vi "attempt-circleFitOnFly.vi"() -> ()   [LabVIEW 2016]
uses:
  <vilib>/vision/Measure.llb/Edge Options.ctl
  <vilib>/vision/Measure.llb/Edge Polarity.ctl
  Motion/HomeMultiple.vi
panel:
  out "Error report":errorcluster
  in  "error in (no error)":errorcluster
  in  "Stop Stage":bool
  out "Moving":bool
  out "Homed":bool
  out "XYZ Stage Current Position":T1={"X [-750, 750 mm]"=-538.7066830444336, "Y [-150, 30 mm]"=-21.699673614501947, "Z [-50, 50 mm]"=3.7042}
  out "N moves":i32
  in  "Send stage to XYZ [mm]":T2
  in  "Axes Speeds [mm/s]":T3={"X Speed"=25.0, "Y Speed"=12.5, "Z Speed"=5.0}
  in  "Home stage":bool
  in  "Move stage":bool
  out "Fitted Circle (Find Circular Edge 1)":T4={"Center (Pixels)"={"X"=1382.2122, "Y"=1051.7542}, "Radius (Pixels)"=145.5667266845703, "Center (Real-World)"={"X"=4111.894, "Y"=-2284.6375}, "Radius (Real-World)"=484.9685191942223, "Roundness (Real-World)"=21.632436942481505, "Average Strength"=60.52941176470587, "Average SNR (dB)"=8.686059708305132} {"Average SNR (dB)" format="%.2f"; "Average Strength" format="%.2f"; "Roundness (Real-World)" format="%.2f"; "Radius (Real-World)" format="%.2f"; "Center (Real-World)"."Y" format="%.2f"; "Center (Real-World)"."X" format="%.2f"; "Radius (Pixels)" format="%.2f"; "Center (Pixels)"."Y" format="%.2f"; "Center (Pixels)"."X" format="%.2f"}
  out "ROI Pixel Statistics (Line Profile 1)":T5={"Min"=5.0, "Max"=255.0, "Mean"=78.77172, "Std Dev"=64.32993, "Count"=2567} {"Min" format="%.2f"; "Std Dev" format="%.2f"; "Mean" format="%.2f"; "Max" format="%.2f"}
  out "Line Profile":cluster{"x0":sgl, "dx":sgl, "Pixels Line":sgl[]}(graph)={"x0"=0.0, "dx"=1.0, "Pixels Line"=[40.0, 43.0, 37.0, 36.0, 39.0, 32.0, 31.0, 26.0, 24.0, 22.0, 19.0, 15.0, 14.0, 14.0, 15.0, 13.0, 11.0, 15.0, 9.0, 15.0, 15.0, 10.0, 9.0, 12.0, 9.0, 9.0, 11.0, 11.0, 10.0, 9.0, 8.0, 8.0, 6.0, 12.0, 9.0, 10.0, 10.0, 7.0, 9.0, 8.0, 12.0, 6.0, 12.0, 10.0, 7.0, 8.0, 7.0, 8.0, 9.0, 8.0, 7.0, 8.0, 10.0, 6.0, 8.0, 10.0, 5.0, 10.0, 8.0, 8.0, 6.0, 8.0, 8.0, 5.0, 7.0, 9.0, 7.0, 7.0, 10.0, 9.0, 8.0, 7.0, 8.0, 10.0, 6.0, 9.0, 9.0, 8.0, 11.0, 11.0, 10.0, 11.0, 12.0, 15.0, 15.0, 15.0, 18.0, 15.0, 19.0, 16.0, 21.0, 22.0, 19.0, 27.0, 23.0, 28.0, 28.0, 33.0, 34.0, 30.0, 42.0, 40.0, 43.0, 44.0, 45.0, 48.0, 48.0, 50.0, 45.0, 48.0, 52.0, 67.0, 57.0, 64.0, 63.0, 61.0, 62.0, 67.0, 65.0, 65.0, 65.0, 73.0, 64.0, 75.0, 74.0, 73.0, 79.0, 77.0, 84.0, 85.0, 87.0, 80.0, 88.0, 86.0, 85.0, 86.0, 91.0, 78.0, 85.0, 83.0, 99.0, 89.0, 95.0, 90.0, 94.0, 87.0, 98.0, 97.0, 99.0, 101.0, 100.0, 96.0, 94.0, 107.0, 106.0, 103.0, 116.0, 109.0, 112.0, 106.0, 105.0, 112.0, 107.0, 113.0, 120.0, 106.0, 114.0, 104.0, 116.0, 119.0, 117.0, 109.0, 117.0, 114.0, 114.0, 112.0, 119.0, 112.0, 117.0, 112.0, 116.0, 123.0, 111.0, 111.0, 115.0, 120.0, 97.0, 112.0, 110.0, 100.0, 113.0, 109.0, 110.0, 116.0, 116.0, 116.0, 112.0, 120.0, 125.0, 106.0, 126.0, 128.0, 113.0, 123.0, 100.0, 106.0, 119.0, 116.0, 123.0, 119.0, 113.0, 128.0, 125.0, 131.0, 133.0, 128.0, 134.0, 137.0, 128.0, 120.0, 122.0, 105.0, 118.0, 111.0, 110.0, 104.0, 105.0, 102.0, 112.0, 100.0, 107.0, 105.0, 114.0, 105.0, 116.0, 104.0, 104.0, 114.0, 106.0, 98.0, 96.0, 89.0, 94.0, 84.0, 88.0, 94.0, 99.0, 94.0, 100.0, 110.0, 112.0, 87.0, 100.0, 94.0, 102.0, 97.0, 107.0, 87.0, 90.0, 93.0, 101.0, 100.0, 104.0, 107.0, 110.0, 100.0, 111.0, 106.0, 104.0, 103.0, 108.0, 101.0, 98.0, 97.0, 98.0, 103.0, 95.0, 99.0, 100.0, 86.0, 97.0, 103.0, 102.0, 102.0, 105.0, 101.0, 102.0, 108.0, 104.0, 97.0, 99.0, 104.0, 103.0, 98.0, 97.0, 104.0, 109.0, 107.0, 109.0, 103.0, 114.0, 114.0, 112.0, 110.0, 102.0, 104.0, 100.0, 98.0, 104.0, 107.0, 107.0, 103.0, 107.0, 101.0, 107.0, 101.0, 105.0, 101.0, 107.0, 89.0, 86.0, 80.0, 79.0, 77.0, 80.0, 85.0, 84.0, 93.0, 88.0, 88.0, 86.0, 89.0, 98.0, 94.0, 93.0, 101.0, 94.0, 108.0, 106.0, 98.0, 106.0, 93.0, 101.0, 98.0, 88.0, 87.0, 85.0, 104.0, 92.0, 87.0, 84.0, 81.0, 89.0, 82.0, 86.0, 81.0, 80.0, 81.0, 84.0, 86.0, 89.0, 89.0, 86.0, 87.0, 86.0, 79.0, 79.0, 88.0, 83.0, 77.0, 84.0, 89.0, 84.0, 85.0, 80.0, 81.0, 80.0, 82.0, 89.0, 95.0, 88.0, 85.0, 90.0, 82.0, 92.0, 94.0, 100.0, 101.0, 89.0, 91.0, 105.0, 103.0, 99.0, 99.0, 100.0, 95.0, 94.0, 97.0, 110.0, 103.0, 103.0, 92.0, 91.0, 98.0, 98.0, 104.0, 95.0, 100.0, 107.0, 101.0, 110.0, 112.0, 104.0, 97.0, 108.0, 107.0, 109.0, 106.0, 116.0, 107.0, 99.0, 104.0, 114.0, 110.0, 109.0, 110.0, 110.0, 113.0, 101.0, 117.0, 108.0, 109.0, 120.0, 103.0, 105.0, 95.0, 91.0, 85.0, 89.0, 89.0, 81.0, 82.0, 79.0, 88.0, 89.0, 90.0, 97.0, 93.0, 104.0, 94.0, 99.0, 105.0, 110.0, 101.0, 97.0, 107.0, 110.0, 91.0, 107.0, 105.0, 119.0, 112.0, 112.0, 112.0, 121.0, 116.0, 131.0, 105.0, 116.0, 113.0, 126.0, 120.0, 115.0, 121.0, 114.0, 111.0, 119.0, 117.0, 121.0, 110.0, 101.0, 113.0, 109.0, 109.0, 111.0, 105.0, 107.0, 109.0, 109.0, 104.0, 107.0, 91.0, 102.0, 112.0, 105.0, 97.0, 103.0, 111.0, 98.0, 103.0, 106.0, 100.0, 111.0, 105.0, 111.0, 109.0, 111.0, 100.0, 104.0, 113.0, 107.0, 113.0, 110.0, 112.0, 95.0, 112.0, 99.0, 108.0, 106.0, 95.0, 98.0, 92.0, 93.0, 88.0, 93.0, 90.0, 88.0, 82.0, 81.0, 80.0, 83.0, 73.0, 78.0, 79.0, 91.0, 92.0, 91.0, 99.0, 105.0, 103.0, 106.0, 104.0, 114.0, 107.0, 101.0, 109.0, 106.0, 107.0, 101.0, 99.0, 98.0, 101.0, 112.0, 107.0, 97.0, 106.0, 108.0, 110.0, 112.0, 104.0, 104.0, 111.0, 103.0, 98.0, 109.0, 104.0, 103.0, 100.0, 104.0, 104.0, 104.0, 102.0, 104.0, 102.0, 104.0, 95.0, 93.0, 91.0, 87.0, 86.0, 88.0, 80.0, 77.0, 80.0, 76.0, 69.0, 69.0, 71.0, 79.0, 83.0, 89.0, 90.0, 86.0, 85.0, 85.0, 81.0, 77.0, 89.0, 85.0, 90.0, 98.0, 96.0, 97.0, 97.0, 105.0, 99.0, 97.0, 104.0, 105.0, 106.0, 101.0, 98.0, 104.0, 93.0, 104.0, 106.0, 101.0, 90.0, 94.0, 107.0, 99.0, 95.0, 92.0, 101.0, 101.0, 98.0, 100.0, 90.0, 92.0, 88.0, 97.0, 98.0, 100.0, 87.0, 101.0, 99.0, 86.0, 100.0, 88.0, 98.0, 97.0, 94.0, 97.0, 99.0, 100.0, 103.0, 98.0, 103.0, 114.0, 107.0, 102.0, 97.0, 99.0, 106.0, 109.0, 112.0, 103.0, 103.0, 103.0, 100.0, 95.0, 99.0, 100.0, 93.0, 94.0, 101.0, 93.0, 97.0, 98.0, 102.0, 95.0, 93.0, 93.0, 106.0, 100.0, 109.0, 98.0, 105.0, 96.0, 101.0, 102.0, 101.0, 92.0, 89.0, 92.0, 86.0, 99.0, 101.0, 94.0, 92.0, 95.0, 95.0, 93.0, 93.0, 92.0, 100.0, 94.0, 85.0, 85.0, 85.0, 85.0, 88.0, 81.0, 94.0, 88.0, 93.0, 100.0, 94.0, 92.0, 88.0, 92.0, 92.0, 95.0, 82.0, 85.0, 88.0, 84.0, 83.0, 94.0, 89.0, 93.0, 88.0, 87.0, 83.0, 91.0, 77.0, 81.0, 85.0, 77.0, 86.0, 89.0, 88.0, 84.0, 80.0, 79.0, 89.0, 89.0, 92.0, 84.0, 94.0, 82.0, 87.0, 90.0, 84.0, 84.0, 92.0, 80.0, 81.0, 71.0, 83.0, 85.0, 87.0, 90.0, 86.0, 93.0, 81.0, 88.0, 91.0, 89.0, 83.0, 95.0, 86.0, 95.0, 90.0, 86.0, 95.0, 84.0, 79.0, 82.0, 85.0, 84.0, 80.0, 82.0, 75.0, 80.0, 89.0, 90.0, 88.0, 85.0, 94.0, 91.0, 93.0, 94.0, 93.0, 88.0, 85.0, 91.0, 82.0, 92.0, 86.0, 84.0, 80.0, 81.0, 88.0, 85.0, 85.0, 93.0, 87.0, 97.0, 94.0, 97.0, 93.0, 97.0, 86.0, 106.0, 92.0, 94.0, 99.0, 101.0, 94.0, 96.0, 89.0, 92.0, 84.0, 89.0, 91.0, 95.0, 103.0, 92.0, 106.0, 104.0, 107.0, 112.0, 97.0, 104.0, 101.0, 104.0, 107.0, 88.0, 91.0, 100.0, 101.0, 102.0, 98.0, 104.0, 104.0, 101.0, 97.0, 98.0, 85.0, 89.0, 98.0, 100.0, 94.0, 95.0, 97.0, 86.0, 95.0, 92.0, 91.0, 98.0, 98.0, 105.0, 94.0, 101.0, 97.0, 88.0, 96.0, 103.0, 109.0, 104.0, 94.0, 88.0, 101.0, 106.0, 93.0, 102.0, 97.0, 95.0, 91.0, 95.0, 87.0, 94.0, 92.0, 101.0, 96.0, 92.0, 93.0, 91.0, 90.0, 92.0, 90.0, 97.0, 95.0, 100.0, 94.0, 106.0, 97.0, 103.0, 94.0, 94.0, 92.0, 101.0, 91.0, 97.0, 85.0, 90.0, 83.0, 83.0, 82.0, 78.0, 73.0, 75.0, 79.0, 74.0, 77.0, 79.0, 78.0, 75.0, 73.0, 77.0, 80.0, 76.0, 69.0, 73.0, 68.0, 70.0, 60.0, 64.0, 55.0, 59.0, 56.0, 53.0, 49.0, 40.0, 39.0, 39.0, 35.0, 28.0, 28.0, 27.0, 23.0, 22.0, 22.0, 25.0, 21.0, 26.0, 19.0, 23.0, 21.0, 21.0, 24.0, 25.0, 22.0, 28.0, 20.0, 18.0, 24.0, 18.0, 18.0, 20.0, 15.0, 16.0, 15.0, 14.0, 13.0, 13.0, 11.0, 13.0, 15.0, 14.0, 18.0, 16.0, 19.0, 15.0, 19.0, 19.0, 18.0, 15.0, 22.0, 15.0, 16.0, 15.0, 16.0, 15.0, 19.0, 16.0, 14.0, 18.0, 16.0, 15.0, 15.0, 15.0, 17.0, 12.0, 18.0, 13.0, 16.0, 12.0, 14.0, 15.0, 10.0, 13.0, 20.0, 15.0, 12.0, 16.0, 18.0, 16.0, 16.0, 17.0, 12.0, 19.0, 15.0, 15.0, 15.0, 13.0, 13.0, 12.0, 15.0, 15.0, 15.0, 17.0, 14.0, 12.0, 15.0, 16.0, 21.0, 11.0, 12.0, 14.0, 17.0, 13.0, 11.0, 17.0, 15.0, 17.0, 17.0, 12.0, 15.0, 18.0, 13.0, 15.0, 17.0, 16.0, 18.0, 17.0, 10.0, 16.0, 16.0, 16.0, 19.0, 14.0, 16.0, 20.0, 14.0, 16.0, 17.0, 15.0, 15.0, 18.0, 16.0, 13.0, 17.0, 13.0, 15.0, 13.0, 21.0, 12.0, 15.0, 14.0, 15.0, 15.0, 15.0, 18.0, 14.0, 14.0, 13.0, 16.0, 16.0, 17.0, 17.0, 15.0, 16.0, 15.0, 15.0, 18.0, 16.0, 15.0, 14.0, 19.0, 16.0, 10.0, 18.0, 13.0, 14.0, 15.0, 15.0, 16.0, 13.0, 15.0, 16.0, 15.0, 13.0, 13.0, 15.0, 14.0, 19.0, 16.0, 17.0, 11.0, 13.0, 12.0, 15.0, 17.0, 20.0, 19.0, 15.0, 22.0, 16.0, 16.0, 15.0, 16.0, 19.0, 15.0, 17.0, 17.0, 15.0, 15.0, 14.0, 16.0, 15.0, 11.0, 17.0, 19.0, 17.0, 14.0, 15.0, 18.0, 18.0, 14.0, 17.0, 18.0, 17.0, 16.0, 18.0, 13.0, 17.0, 18.0, 15.0, 12.0, 20.0, 17.0, 15.0, 16.0, 19.0, 17.0, 21.0, 13.0, 15.0, 20.0, 16.0, 16.0, 17.0, 18.0, 16.0, 21.0, 16.0, 16.0, 19.0, 19.0, 20.0, 16.0, 22.0, 19.0, 20.0, 16.0, 18.0, 16.0, 19.0, 17.0, 22.0, 18.0, 15.0, 18.0, 19.0, 15.0, 21.0, 17.0, 17.0, 19.0, 19.0, 21.0, 15.0, 21.0, 17.0, 24.0, 18.0, 20.0, 17.0, 17.0, 21.0, 19.0, 17.0, 19.0, 21.0, 18.0, 21.0, 17.0, 18.0, 28.0, 24.0, 24.0, 22.0, 29.0, 36.0, 39.0, 49.0, 52.0, 66.0, 99.0, 142.0, 181.0, 219.0, 214.0, 193.0, 195.0, 163.0, 173.0, 193.0, 230.0, 246.0, 255.0, 255.0, 255.0, 255.0, 255.0, 255.0, 255.0, 255.0, 255.0, 255.0, 255.0, 255.0, 255.0, 255.0, 255.0, 255.0, 255.0, 248.0, 240.0, 222.0, 220.0, 211.0, 219.0, 212.0, 219.0, 219.0, 216.0, 217.0, 207.0, 216.0, 228.0, 215.0, 227.0, 211.0, 226.0, 221.0, 207.0, 222.0, 245.0, 239.0, 253.0, 255.0, 255.0, 255.0, 255.0, 255.0, 255.0, 255.0, 255.0, 255.0, 255.0, 255.0, 255.0, 255.0, 255.0, 255.0, 255.0, 255.0, 255.0, 255.0, 255.0, 255.0, 255.0, 255.0, 255.0, 255.0, 255.0, 255.0, 255.0, 255.0, 255.0, 255.0, 255.0, 255.0, 255.0, 255.0, 255.0, 255.0, 255.0, 255.0, 255.0, 255.0, 255.0, 240.0, 198.0, 182.0, 179.0, 193.0, 200.0, 216.0, 202.0, 196.0, 199.0, 195.0, 210.0, 214.0, 253.0, 255.0, 255.0, 255.0, 255.0, 255.0, 255.0, 248.0, 234.0, 251.0, 255.0, 255.0, 255.0, 255.0, 255.0, 255.0, 255.0, 255.0, 255.0, 255.0, 255.0, 255.0, 255.0, 255.0, 252.0, 217.0, 205.0, 207.0, 233.0, 217.0, 230.0, 239.0, 228.0, 211.0, 199.0, 207.0, 205.0, 213.0, 215.0, 217.0, 217.0, 204.0, 229.0, 232.0, 230.0, 222.0, 233.0, 254.0, 255.0, 255.0, 255.0, 244.0, 233.0, 206.0, 229.0, 194.0, 205.0, 197.0, 179.0, 187.0, 185.0, 205.0, 223.0, 239.0, 246.0, 255.0, 255.0, 255.0, 255.0, 254.0, 230.0, 216.0, 197.0, 192.0, 210.0, 181.0, 198.0, 192.0, 202.0, 212.0, 226.0, 247.0, 240.0, 229.0, 223.0, 233.0, 255.0, 255.0, 255.0, 247.0, 230.0, 216.0, 218.0, 226.0, 255.0, 255.0, 253.0, 255.0, 255.0, 237.0, 247.0, 244.0, 248.0, 255.0, 255.0, 255.0, 255.0, 250.0, 243.0, 220.0, 215.0, 218.0, 226.0, 242.0, 255.0, 255.0, 255.0, 255.0, 255.0, 255.0, 255.0, 255.0, 255.0, 255.0, 255.0, 255.0, 248.0, 255.0, 255.0, 255.0, 210.0, 190.0, 166.0, 158.0, 163.0, 189.0, 200.0, 214.0, 207.0, 192.0, 201.0, 199.0, 190.0, 172.0, 165.0, 166.0, 176.0, 171.0, 192.0, 189.0, 178.0, 162.0, 168.0, 166.0, 178.0, 181.0, 191.0, 190.0, 178.0, 162.0, 167.0, 163.0, 173.0, 162.0, 163.0, 157.0, 159.0, 158.0, 158.0, 159.0, 174.0, 190.0, 190.0, 209.0, 217.0, 230.0, 252.0, 244.0, 247.0, 232.0, 223.0, 210.0, 179.0, 175.0, 128.0, 99.0, 58.0, 49.0, 38.0, 33.0, 28.0, 23.0, 23.0, 31.0, 19.0, 27.0, 18.0, 17.0, 18.0, 15.0, 21.0, 18.0, 15.0, 18.0, 16.0, 15.0, 17.0, 14.0, 18.0, 22.0, 14.0, 16.0, 19.0, 13.0, 18.0, 18.0, 14.0, 14.0, 14.0, 16.0, 16.0, 16.0, 16.0, 15.0, 17.0, 14.0, 19.0, 15.0, 17.0, 17.0, 16.0, 15.0, 12.0, 19.0, 19.0, 19.0, 18.0, 12.0, 20.0, 17.0, 16.0, 13.0, 15.0, 17.0, 16.0, 19.0, 17.0, 15.0, 15.0, 14.0, 19.0, 13.0, 20.0, 19.0, 18.0, 23.0, 15.0, 12.0, 17.0, 20.0, 13.0, 14.0, 13.0, 12.0, 16.0, 18.0, 17.0, 19.0, 19.0, 17.0, 13.0, 18.0, 18.0, 16.0, 16.0, 19.0, 17.0, 18.0, 18.0, 18.0, 13.0, 17.0, 14.0, 16.0, 14.0, 15.0, 11.0, 12.0, 16.0, 15.0, 11.0, 16.0, 16.0, 17.0, 16.0, 12.0, 20.0, 16.0, 16.0, 16.0, 15.0, 15.0, 13.0, 19.0, 16.0, 15.0, 11.0, 17.0, 15.0, 20.0, 8.0, 15.0, 16.0, 19.0, 16.0, 16.0, 14.0, 17.0, 16.0, 20.0, 15.0, 20.0, 18.0, 15.0, 17.0, 21.0, 20.0, 16.0, 21.0, 20.0, 21.0, 17.0, 23.0, 18.0, 15.0, 13.0, 15.0, 12.0, 9.0, 14.0, 14.0, 15.0, 11.0, 13.0, 12.0, 14.0, 13.0, 17.0, 15.0, 13.0, 12.0, 12.0, 18.0, 16.0, 13.0, 11.0, 16.0, 18.0, 14.0, 16.0, 17.0, 15.0, 12.0, 16.0, 18.0, 16.0, 14.0, 18.0, 15.0, 19.0, 13.0, 13.0, 18.0, 13.0, 13.0, 14.0, 12.0, 12.0, 14.0, 16.0, 15.0, 13.0, 14.0, 13.0, 11.0, 15.0, 15.0, 19.0, 18.0, 18.0, 15.0, 16.0, 17.0, 15.0, 15.0, 18.0, 13.0, 16.0, 18.0, 18.0, 17.0, 16.0, 19.0, 29.0, 29.0, 41.0, 52.0, 61.0, 65.0, 84.0, 92.0, 89.0, 101.0, 101.0, 99.0, 112.0, 113.0, 104.0, 107.0, 113.0, 116.0, 114.0, 114.0, 113.0, 120.0, 130.0, 136.0, 153.0, 162.0, 164.0, 174.0, 183.0, 181.0, 171.0, 168.0, 168.0, 163.0, 148.0, 149.0, 138.0, 132.0, 126.0, 127.0, 107.0, 117.0, 113.0, 120.0, 119.0, 114.0, 100.0, 110.0, 100.0, 107.0, 111.0, 98.0, 97.0, 97.0, 88.0, 87.0, 91.0, 95.0, 85.0, 88.0, 90.0, 86.0, 83.0, 84.0, 81.0, 82.0, 82.0, 85.0, 88.0, 87.0, 79.0, 68.0, 67.0, 64.0, 72.0, 68.0, 68.0, 75.0, 70.0, 88.0, 76.0, 87.0, 75.0, 81.0, 77.0, 90.0, 85.0, 89.0, 99.0, 92.0, 96.0, 95.0, 109.0, 94.0, 86.0, 93.0, 86.0, 80.0, 83.0, 86.0, 90.0, 94.0, 89.0, 97.0, 95.0, 104.0, 97.0, 107.0, 101.0, 101.0, 94.0, 92.0, 100.0, 95.0, 94.0, 89.0, 95.0, 83.0, 87.0, 88.0, 76.0, 83.0, 92.0, 93.0, 93.0, 95.0, 98.0, 97.0, 99.0, 89.0, 96.0, 97.0, 93.0, 94.0, 96.0, 85.0, 92.0, 92.0, 87.0, 99.0, 93.0, 90.0, 96.0, 98.0, 88.0, 92.0, 97.0, 99.0, 98.0, 92.0, 91.0, 86.0, 87.0, 100.0, 93.0, 86.0, 87.0, 83.0, 75.0, 80.0, 73.0, 62.0, 73.0, 65.0, 67.0, 68.0, 79.0, 74.0, 70.0, 75.0, 70.0, 72.0, 65.0, 65.0, 66.0, 67.0, 69.0, 73.0, 74.0, 69.0, 76.0, 79.0, 71.0, 74.0, 72.0, 79.0, 76.0, 74.0, 72.0, 74.0, 71.0, 68.0, 71.0, 71.0, 85.0, 85.0, 81.0, 88.0, 79.0, 84.0, 84.0, 80.0, 80.0, 83.0, 85.0, 80.0, 89.0, 97.0, 92.0, 83.0, 84.0, 92.0, 82.0, 81.0, 91.0, 85.0, 83.0, 89.0, 82.0, 93.0, 85.0, 86.0, 89.0, 86.0, 87.0, 76.0, 79.0, 80.0, 72.0, 77.0, 70.0, 76.0, 85.0, 80.0, 74.0, 73.0, 80.0, 73.0, 82.0, 64.0, 71.0, 64.0, 64.0, 68.0, 67.0, 71.0, 63.0, 75.0, 67.0, 71.0, 67.0, 62.0, 66.0, 60.0, 67.0, 68.0, 63.0, 69.0, 68.0, 67.0, 68.0, 58.0, 67.0, 64.0, 58.0, 61.0, 58.0, 54.0, 60.0, 62.0, 68.0, 58.0, 62.0, 57.0, 64.0, 71.0, 70.0, 68.0, 68.0, 63.0, 73.0, 73.0, 65.0, 55.0, 52.0, 45.0, 40.0, 42.0, 48.0, 52.0, 53.0, 51.0, 56.0, 56.0, 56.0, 51.0, 53.0, 61.0, 59.0, 54.0, 51.0, 46.0, 44.0, 45.0, 50.0, 47.0, 50.0, 44.0, 47.0, 57.0, 54.0, 58.0, 55.0, 68.0, 57.0, 72.0, 62.0, 61.0, 65.0, 73.0, 65.0, 67.0, 69.0, 71.0, 71.0, 73.0, 62.0, 69.0, 67.0, 66.0, 69.0, 64.0, 70.0, 69.0, 73.0, 81.0, 71.0, 77.0, 77.0, 67.0, 72.0, 75.0, 72.0, 72.0, 74.0, 76.0, 72.0, 81.0, 74.0, 74.0, 87.0, 79.0, 65.0, 83.0, 70.0, 77.0, 70.0, 74.0, 74.0, 86.0, 79.0, 73.0, 70.0, 64.0, 69.0, 70.0, 79.0, 75.0, 77.0, 68.0, 71.0, 64.0, 64.0, 77.0, 74.0, 69.0, 72.0, 73.0, 64.0, 64.0, 66.0, 60.0, 66.0, 66.0, 62.0, 64.0, 64.0, 68.0, 64.0, 62.0, 64.0, 64.0, 67.0, 70.0, 63.0, 60.0, 67.0, 63.0, 65.0, 67.0, 72.0, 64.0, 67.0, 67.0, 64.0, 54.0, 57.0, 53.0, 62.0, 62.0, 64.0, 68.0, 64.0, 70.0, 65.0, 79.0, 76.0, 71.0, 68.0, 66.0, 50.0, 46.0, 45.0, 39.0, 46.0, 40.0, 44.0, 46.0, 48.0, 59.0, 55.0, 58.0, 56.0, 58.0, 60.0, 55.0, 52.0, 56.0, 54.0, 55.0, 54.0, 59.0, 57.0, 70.0, 71.0, 79.0, 69.0, 60.0, 56.0, 56.0, 49.0, 40.0, 36.0, 44.0, 41.0, 37.0, 33.0, 43.0, 41.0, 56.0, 57.0, 52.0, 50.0, 47.0, 45.0, 43.0, 51.0, 50.0, 47.0, 56.0, 55.0, 53.0, 55.0, 49.0, 52.0, 53.0, 55.0, 48.0, 55.0, 48.0, 46.0, 51.0, 55.0, 56.0, 60.0, 53.0, 39.0, 36.0, 39.0, 36.0, 37.0, 34.0, 32.0, 35.0, 33.0, 32.0, 37.0, 43.0, 39.0, 44.0, 44.0, 43.0, 42.0, 44.0, 46.0, 42.0, 37.0, 39.0, 36.0, 38.0, 31.0, 34.0, 30.0, 34.0, 31.0, 35.0, 40.0, 34.0, 31.0, 32.0, 31.0, 34.0, 30.0, 38.0, 34.0, 32.0, 33.0, 34.0, 33.0, 39.0, 33.0, 39.0, 36.0, 33.0, 27.0, 25.0, 25.0, 22.0, 20.0, 28.0, 26.0, 31.0, 29.0, 32.0, 37.0, 36.0, 30.0, 24.0, 25.0, 30.0, 21.0, 23.0, 27.0, 22.0, 25.0, 27.0, 27.0, 29.0, 26.0, 22.0, 29.0, 28.0, 23.0, 26.0, 27.0, 28.0, 27.0, 31.0, 24.0, 25.0, 30.0, 34.0, 29.0, 28.0, 31.0, 31.0, 31.0, 32.0, 39.0, 34.0, 33.0, 27.0, 24.0, 22.0, 22.0, 23.0, 21.0, 29.0, 27.0, 30.0, 24.0, 23.0, 28.0, 23.0, 31.0, 29.0, 28.0, 27.0, 27.0, 25.0, 27.0, 33.0, 40.0, 32.0, 36.0, 35.0, 35.0, 31.0, 24.0, 31.0, 21.0, 25.0, 23.0, 24.0, 28.0, 24.0, 21.0, 25.0, 26.0, 25.0, 32.0, 30.0, 37.0, 39.0, 40.0, 39.0, 36.0, 28.0, 25.0, 22.0, 22.0, 26.0, 26.0, 25.0, 25.0, 27.0, 28.0, 32.0, 30.0, 31.0, 28.0, 36.0, 37.0, 34.0, 36.0, 34.0, 36.0, 32.0, 30.0, 31.0, 27.0, 27.0, 24.0, 27.0, 22.0, 24.0, 27.0, 24.0, 30.0, 33.0, 29.0, 26.0, 30.0, 31.0, 26.0, 31.0, 28.0, 32.0, 24.0, 27.0, 33.0, 25.0, 28.0, 33.0, 35.0, 36.0, 34.0, 25.0, 24.0, 24.0, 25.0, 24.0, 28.0, 24.0, 33.0, 27.0, 29.0, 30.0, 26.0, 29.0, 29.0, 30.0, 28.0, 26.0, 22.0, 19.0, 30.0, 29.0, 24.0, 21.0, 25.0, 25.0, 30.0, 24.0, 21.0, 19.0, 25.0, 22.0, 18.0, 24.0, 19.0, 23.0, 19.0, 20.0, 19.0, 18.0, 22.0, 21.0, 17.0, 19.0, 20.0, 18.0, 18.0, 18.0, 19.0, 17.0, 19.0, 13.0, 19.0, 13.0, 22.0, 19.0, 19.0, 18.0, 16.0, 19.0, 18.0, 21.0, 17.0, 19.0, 21.0, 16.0, 19.0, 16.0, 19.0, 20.0, 18.0, 16.0, 14.0, 15.0, 20.0, 19.0, 16.0, 19.0, 19.0, 15.0, 22.0, 20.0, 18.0, 20.0, 23.0, 18.0, 22.0, 21.0, 18.0, 22.0, 23.0, 19.0, 24.0, 22.0, 22.0, 25.0, 23.0, 23.0, 19.0, 21.0, 21.0, 27.0, 28.0, 30.0, 27.0, 31.0, 28.0, 24.0, 25.0, 28.0, 30.0, 36.0, 36.0, 32.0, 31.0, 28.0, 34.0, 31.0, 35.0, 36.0, 37.0, 35.0, 39.0, 30.0, 30.0, 33.0, 29.0, 31.0, 34.0, 37.0, 38.0, 44.0, 35.0, 39.0, 34.0, 34.0, 37.0, 30.0, 39.0, 30.0, 35.0, 30.0, 32.0, 34.0, 33.0, 35.0, 35.0, 34.0, 30.0, 36.0, 30.0, 30.0, 25.0, 23.0, 24.0, 22.0, 18.0, 20.0, 15.0, 15.0, 13.0, 10.0, 11.0, 10.0, 8.0, 8.0, 5.0, 8.0, 6.0, 5.0]}
  in  "Circle Fit Options":T6={"Process"=enum."Get First Edge", "Step Size"=10, "Max Pixel Radius"=3}
  in  "Options (Find Circular Edge 1)":T9={"Search  Direction"=0, "Edge Options"={"Edge Polarity"=0, "Kernel Size"=3, "Width"=3, "Minimum Edge Strength"=50.0, "Interpolation Type"=enum."Bilinear Fixed", "Data Processing Method"=enum."Average"}, "Show Search Area"=TRUE, "Show Search Lines"=TRUE, "Show Edges Found"=TRUE, "Show Result"=TRUE, "Search Area Color"=65280, "Search Lines Color"=255, "Edge Locations Color"=16776960, "Result Color"=16711680, "Overlay Group Name"=""} {"Search  Direction" items=["Outside to Inside", "Inside to Outside"]; "Edge Options"."Edge Polarity" items=["All Edges", "Rising Edges", "Falling Edges"]; "Edge Options"."Minimum Edge Strength" format="%.2f"; "Edge Options"."Width" step=2; "Edge Options"."Kernel Size" step=2}
  out "Image Number":u32=372
  in  "Stop Camera":bool
  out "Image Out":T10(plugin-control)
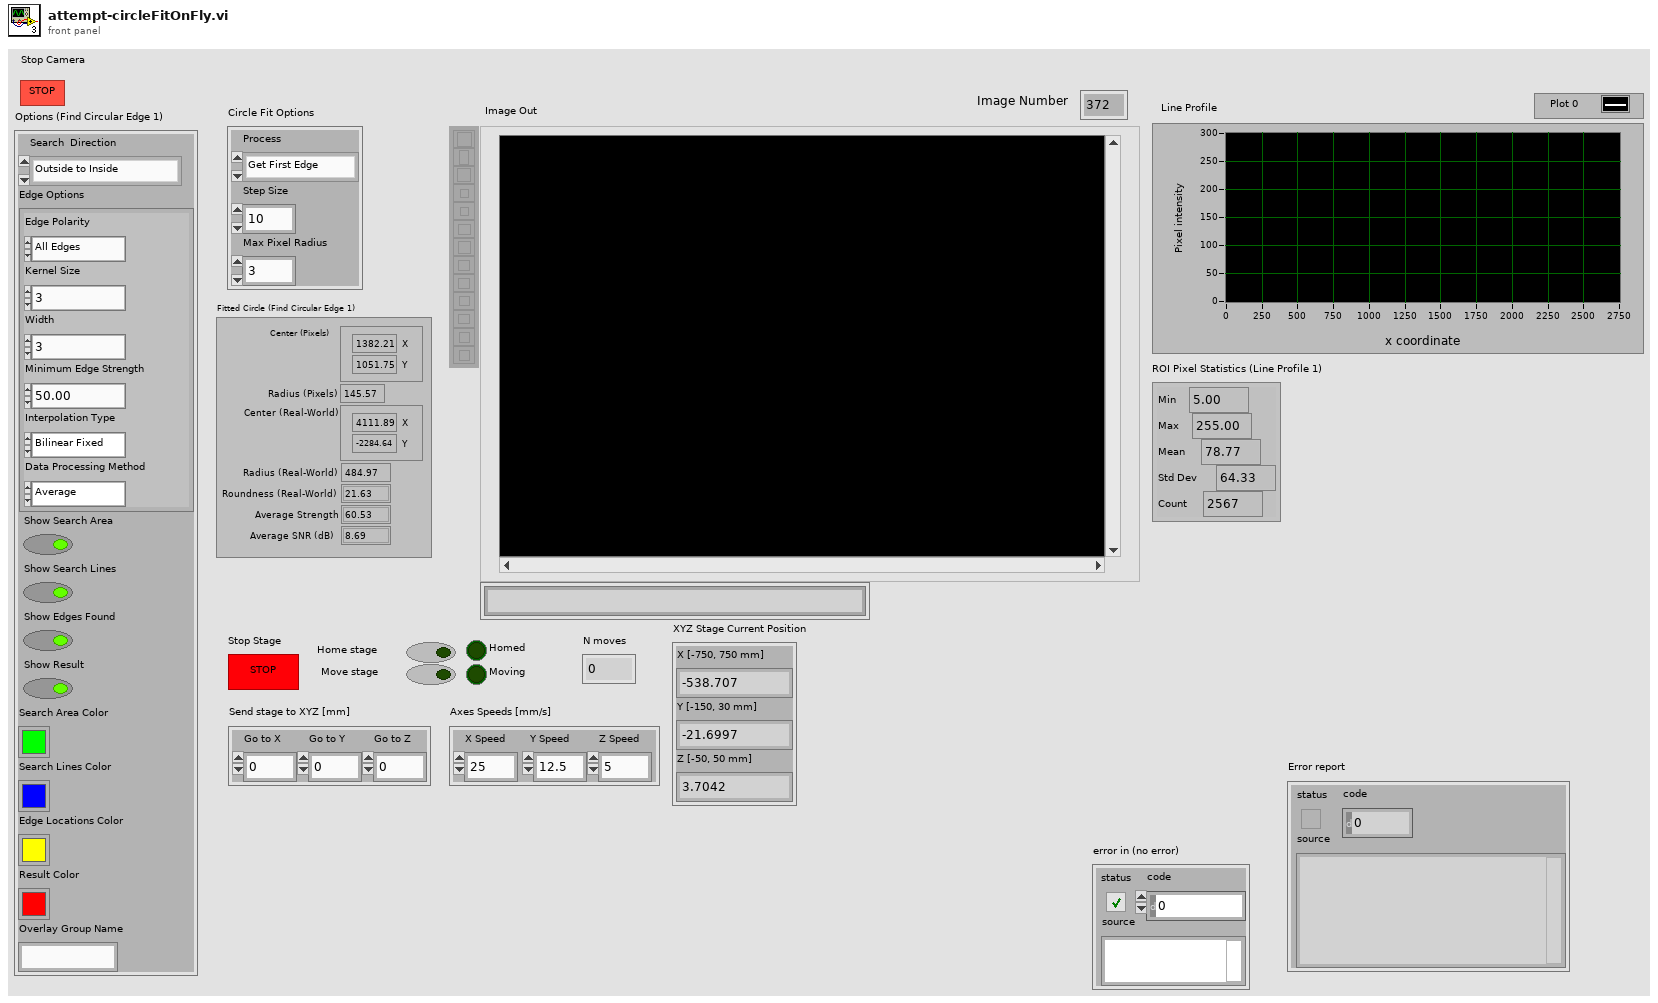
[diagram p1: front panel]
types:
  T1 = cluster{"X [-750, 750 mm]":dbl, "Y [-150, 30 mm]":dbl, "Z [-50, 50 mm]":dbl}
  T2 = cluster{"Go to X":dbl, "Go to Y":dbl, "Go to Z":dbl}
  T3 = cluster{"X Speed":dbl, "Y Speed":dbl, "Z Speed":dbl}
  T4 = cluster{"Center (Pixels)":cluster{"X":sgl, "Y":sgl}, "Radius (Pixels)":dbl, "Center (Real-World)":cluster{"X":sgl, "Y":sgl}, "Radius (Real-World)":dbl, "Roundness (Real-World)":dbl, "Average Strength":dbl, "Average SNR (dB)":dbl}
  T5 = cluster{"Min":sgl, "Max":sgl, "Mean":sgl, "Std Dev":sgl, "Count":i32}
  T6 = cluster{"Process":enum16{"Get First Edge", "Get First + Last Edge", "Get All Edges", "Get Best Edge"}, "Step Size":i32, "Max Pixel Radius":i32}
  T7 = typedef "Edge Options.ctl" = cluster{"Edge Polarity":T8, "Kernel Size":u32, "Width":u32, "Minimum Edge Strength":sgl, "Interpolation Type":enum32{"Zero Order", "Bilinear", "Quadratic", "Cubic", "Bilinear Fixed"}, "Data Processing Method":enum32{"Average", "Median"}}
  T8 = typedef "Edge Polarity.ctl" = u32
  T9 = cluster{"Search  Direction":u32, "Edge Options":T7, "Show Search Area":bool, "Show Search Lines":bool, "Show Edges Found":bool, "Show Result":bool, "Search Area Color":u32, "Search Lines Color":u32, "Edge Locations Color":u32, "Result Color":u32, "Overlay Group Name":string}
  T10 = typedef "IMAQ Image.ctl" = refnum<image>
  T11 = cluster{"Program Position Feedback":dbl, "Program Position Feedback 2":dbl, "Program Position Feedback 3":dbl}
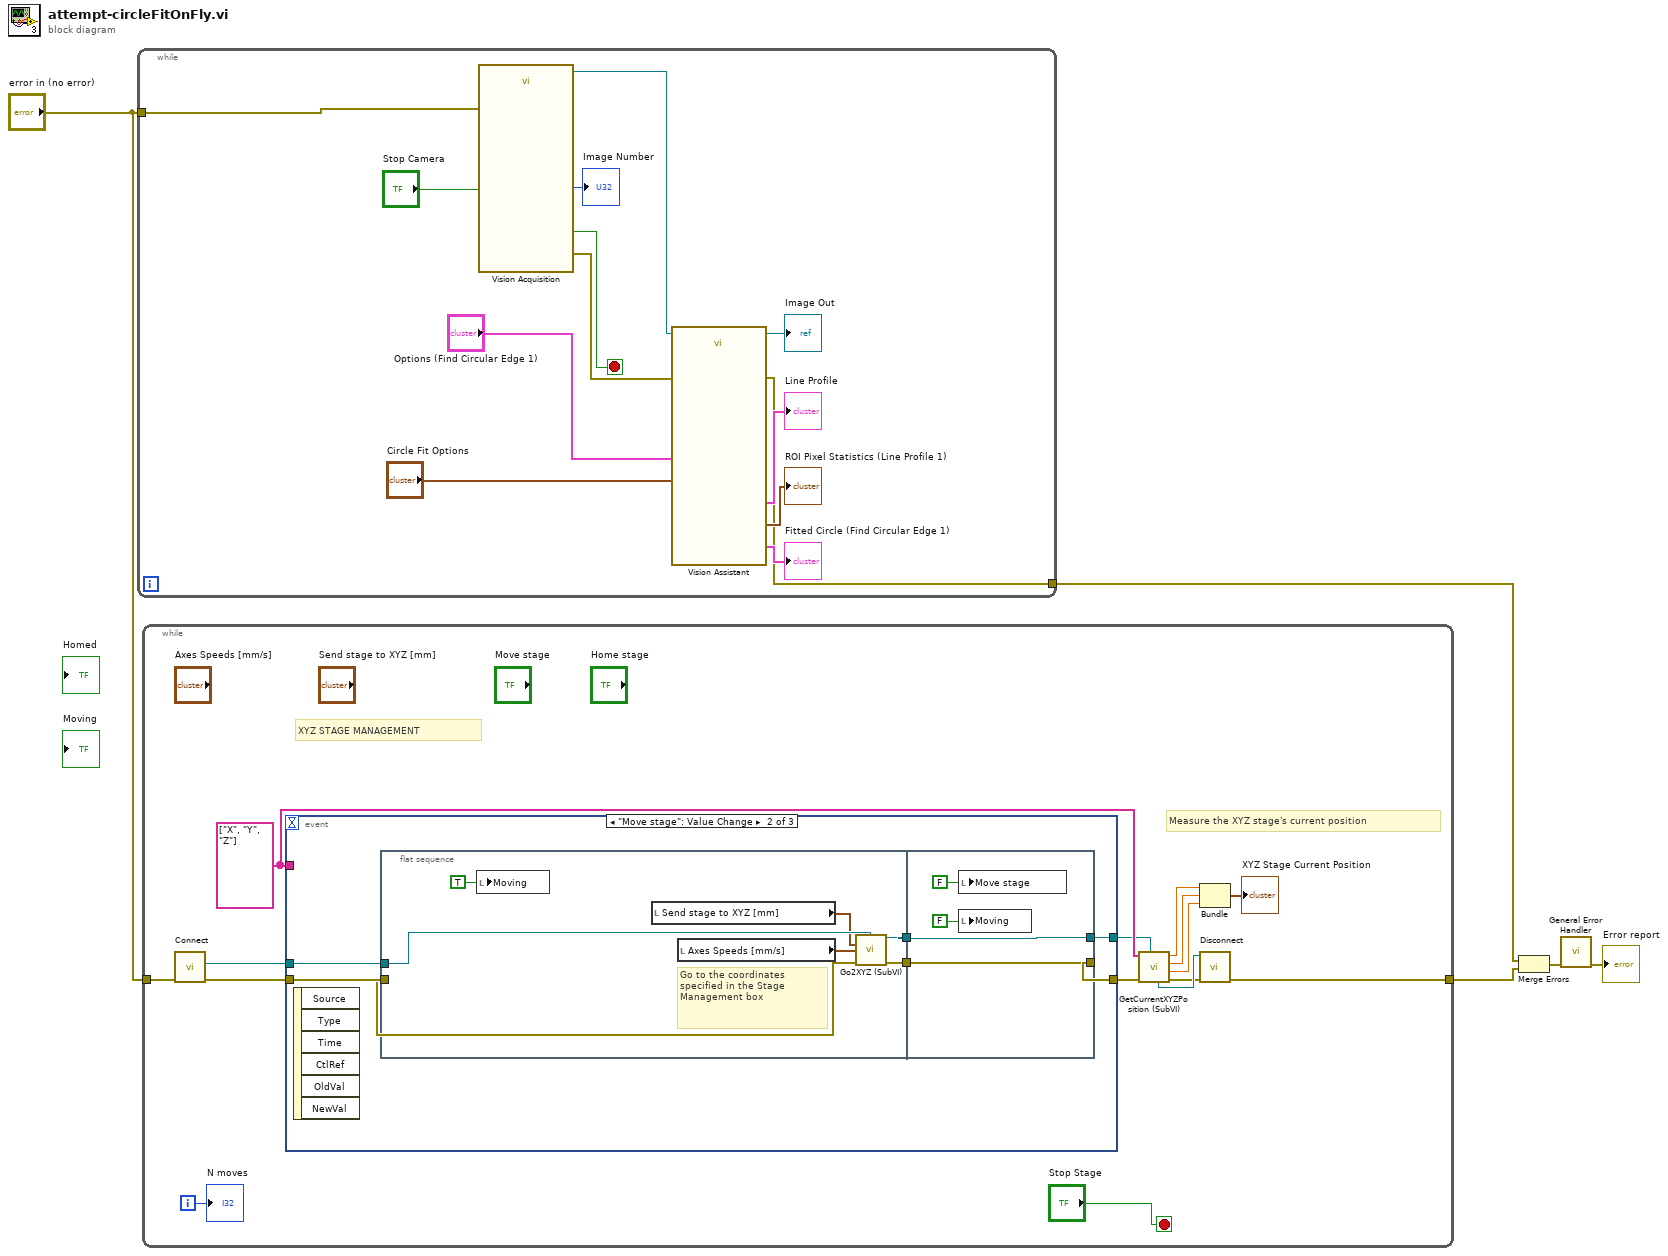
[diagram p0: block diagram]
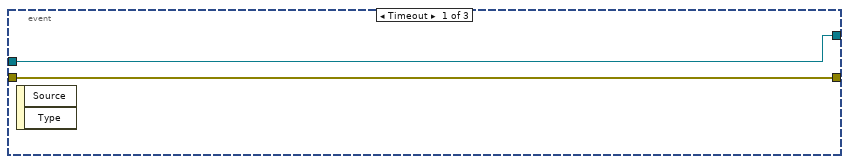
[diagram p2: hidden frame]
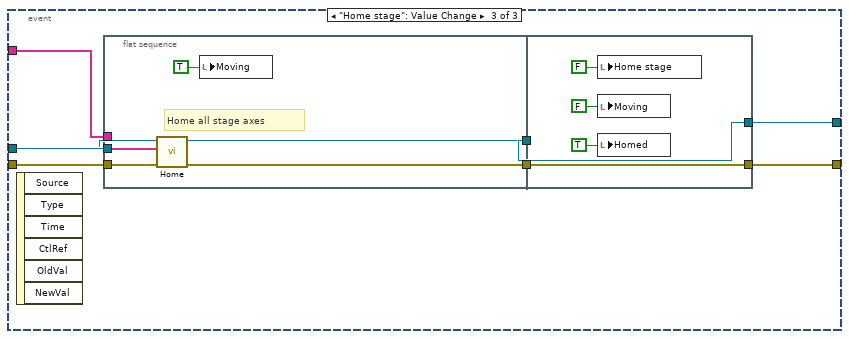
[diagram p3: hidden frame]
diagram:
  n1 = while {
    tunnel: "error in (no error)" -> [w8]
    tunnel: [w6] -> w3
    stop <- w17 stop-if-true
    n2 = call "Vision Acquisition"("Stop (F)"="Stop Camera", "error in"=w8) -> ("Image Out"=w15:T10, "Image Number"=→"Image Number":u32, "Stopped"=w17:bool, "error out"=w7:errorcluster)  [unwired: 21 in, 1 out]
    n3 = call "Vision Assistant"("Image In"=w15, "Options (Find Circular Edge 1)"="Options (Find Circular Edge 1)", "Circle Fit Options (Find Circular Edge 1)"="Circle Fit Options", "error in"=w7) -> ("Image Out"=→"Image Out":T10, "Line Profile (Line Profile 1)"=→"Line Profile":cluster{"x0":sgl, "dx":sgl, "Pixels Line":sgl[]}, "ROI Pixel Statistics (Line Profile 1)"=→"ROI Pixel Statistics (Line Profile 1)":T5, "Fitted Circle (Find Circular Edge 1)"=→"Fitted Circle (Find Circular Edge 1)":T4, "error out"=w6:errorcluster)  [unwired: 19 in]
  }
  n4 = while {
    tunnel: "error in (no error)" -> [w33]
    tunnel: [w20] -> w1
    i -> [w23]
    stop <- "Stop Stage" stop-if-true
    w24 = string[] ["X", "Y", "Z"] ("Axes Names")
    # "XYZ STAGE MANAGEMENT"
    # "Measure the XYZ stage's current position"
    n5 = call "Connect.vi"("error in (no error)"=w33) -> ("error out"=w31:errorcluster, "controller"=w32:refnum<k24>)  [unwired: 9 in]
    n6 = event shown="[1] \"Move stage\": Value Change" {
      selector: _ -> [_ _ _]
      dyn-events: _ -> [_ _ _]
      timeout: _ -> [_ _ _]
      tunnel: w32 -> [w35 w41 w59]
      tunnel: w31 -> [w34 w38 w58]
      tunnel: [w35 w40 w56] -> w22
      tunnel: [w34 w39 w57] -> w25
      tunnel: w24 -> [_ _ w55]
      event Timeout {
        n7 = event-data() -> ()  [unwired: 1 in, 2 out]
      }
      event "Move stage": Value Change {
        n8 = event-data() -> ()  [unwired: 1 in, 6 out]
        n9 = flat-sequence {
          tunnel: w41 -> [w48]
          tunnel: w38 -> [w45]
          tunnel: [w47] -> w37
          tunnel: [w46] -> w36
          tunnel: [w51] -> w39
          tunnel: [w52] -> w40
          tunnel: w37 -> [w52]
          tunnel: w36 -> [w51]
          frame #0 {
            # "Go to the coordinates\nspecified in the Stage\nManagement box"
            n10 = local write "Moving"(TRUE ("Moving")) -> ()
            n11 = local read "Send stage to XYZ [mm]"() -> (w43:T2)
            n12 = local read "Axes Speeds [mm/s]"() -> (w42:T3)
            n13 = call "Go2XYZ (SubVI).vi"(".NET Refnum in"=w48, "Go to Coordinates"=w43, "Axis Speeds"=w42, "error in (no error)"=w45) -> (".NET Refnum out"=w47:refnum<k24>, "error out"=w46:errorcluster)  [unwired: 8 in, 2 out]
          }
          frame #1 {
            n14 = local write "Move stage"(FALSE ("Move stage")) -> ()
            n15 = local write "Moving"(FALSE ("Moving")) -> ()
          }
        }
      }
      event "Home stage": Value Change {
        n16 = event-data() -> ()  [unwired: 1 in, 6 out]
        n17 = flat-sequence {
          tunnel: w59 -> [w65]
          tunnel: w58 -> [w64]
          tunnel: w55 -> [w61]
          tunnel: [w63] -> w54
          tunnel: [w62] -> w53
          tunnel: [w69] -> w56
          tunnel: [w70] -> w57
          tunnel: w54 -> [w70]
          tunnel: w53 -> [w69]
          frame #0 {
            # "Home all stage axes"
            n18 = call-poly "Home.vi"("error in (no error)"=w64, "axis names"=w61, "controller in"=w65) -> ("error out"=w63:errorcluster, "controller out"=w62:refnum<k24>)  [unwired: 7 in]
            n19 = local write "Moving"(TRUE ("Moving")) -> ()
          }
          frame #1 {
            n20 = local write "Home stage"(FALSE ("Home stage")) -> ()
            n21 = local write "Moving"(FALSE ("Moving")) -> ()
            n22 = local write "Homed"(TRUE ("Homed")) -> ()
          }
        }
      }
    }
    n23 = call "GetCurrentXYZPosition (SubVI).vi"(".NET Refnum in - Device"=w22, "error in (no error)"=w25, "Axes Names"=w24) -> ("error out"=w21:errorcluster, "Program Position Feedback 3"=w30:dbl, "Program Position Feedback 2"=w29:dbl, "Program Position Feedback"=w28:dbl, ".NET Refnum out  - Device"=w27:refnum<k24>)  [unwired: 3 in]
    n24 = Bundle("Program Position Feedback"=w28, "Program Position Feedback 2"=w29, "Program Position Feedback 3"=w30) -> (→"XYZ Stage Current Position":T11)  [unwired: 1 in]
    n25 = call "Disconnect.vi"("error in (no error)"=w21, "controller"=w27) -> ("error out"=w20:errorcluster)  [unwired: 9 in]
    "N moves" <- w23
  }
  n26 = Merge Errors(w3, w1) -> (w4:errorcluster)
  n27 = call <vilib>:"General Error Handler.vi"("error in (no error)"=w4) -> ("error out"=→"Error report":errorcluster)  [unwired: 2 in, 12 out]
